vi "test_work(4800).vi"() -> ()   [LabVIEW 2013]
uses:
  IS-95/receiver/4800/Combination device(4800).vi
  IS-95/receiver/common/Path Searcher.vi
  IS-95/transmitter/4800/coding(4800).vi
  IS-95/transmitter/common/interleaver.vi
  IS-95/transmitter/9600/coding(9600).vi
  <vilib>/Analysis/baseanly.llb/A x B.vi
  <vilib>/Analysis/baseanly.llb/Real A x B.vi
  IS-95/receiver/common/Viterbi.vi
  IS-95/receiver/4800/FER(4800).vi
  IS-95/receiver/common/Peak detection.vi
  IS-95/transmitter/4800/syndrom(4800).vi
  IS-95/transmitter/9600/syndrom(9600).vi
  IS-95/receiver/common/metrics.vi
  <vilib>/Analysis/Matrix/Numeric/Conversions/Array To Matrix.vi
  <vilib>/Analysis/Matrix/Numeric/Conversions/Array To Matrix - RA.vi
  <vilib>/ptbypt/Other Functions.llb/Complex Queue PtByPt.vi
  <vilib>/ptbypt/Time Domain.llb/Peak Detector PtByPt.vi
  IS-95/receiver/4800/Gateway(4800).vi
panel:
  in  "Stop Button":bool
  out "ПЕРЕДАЧА":bool[](array[boolean])
  in  "ПЕРЕДАЧА":u16(ring)=2 items=["0", "1", "2", "3", "4", "5", "6", "7", "8", "9", "10", "11", "12", "13", "14", "15", "16", "17", "18", "19", "20", "21", "22", "23", "24", "25", "26", "27", "28", "29", "30", "31", "32", "33", "34", "35", "36", "37", "38", "39", "40", "41", "42", "43", "44", "45", "46", "47", "48", "49", "50", "51", "52", "53", "54", "55", "56", "57", "58", "59", "60", "61", "62", "63"]
  in  "ПРИЕМ":u16(ring)=2 items=["0", "1", "2", "3", "4", "5", "6", "7", "8", "9", "10", "11", "12", "13", "14", "15", "16", "17", "18", "19", "20", "21", "22", "23", "24", "25", "26", "27", "28", "29", "30", "31", "32", "33", "34", "35", "36", "37", "38", "39", "40", "41", "42", "43", "44", "45", "46", "47", "48", "49", "50", "51", "52", "53", "54", "55", "56", "57", "58", "59", "60", "61", "62", "63"]
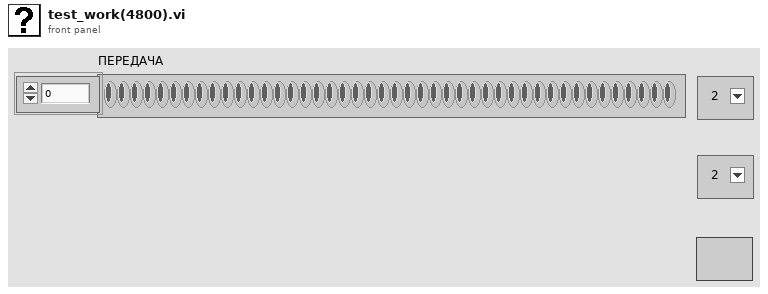
[diagram p1: front panel]
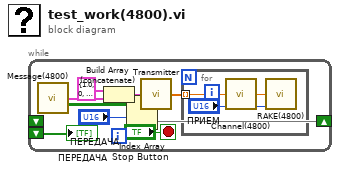
[diagram p0: block diagram]
diagram:
  n1 = while {
    shift-right: [w2] -> _
    shift-left: _ -> [_]
    shift-left: _ -> [w1]
    stop <- "Stop Button" stop-if-true
    n2 = call "Message(4800).vi"() -> ("Channels"=w5:cluster{dbl, i32, bool[], "Type":i32}[], "Message"=w4:bool[][])  [unwired: 14 in]
    n3 = Build Array (concatenate)(cluster{dbl, i32, bool[], "Type":i32} {1.0, 0, [FALSE, FALSE, FALSE, FALSE, FALSE, FALSE, FALSE, FALSE, FALSE, FALSE, FALSE, FALSE, FALSE, FALSE, FALSE, FALSE, FALSE, FALSE, FALSE, FALSE, FALSE, FALSE, FALSE, FALSE, FALSE, FALSE, FALSE, FALSE, FALSE, FALSE, FALSE, FALSE, FALSE, FALSE, FALSE, FALSE, FALSE, FALSE, FALSE, FALSE, FALSE, FALSE, FALSE, FALSE, FALSE, FALSE, FALSE, FALSE, FALSE, FALSE, FALSE, FALSE, FALSE, FALSE, FALSE, FALSE, FALSE, FALSE, FALSE, FALSE, FALSE, FALSE, FALSE, FALSE, FALSE, FALSE, FALSE, FALSE, FALSE, FALSE, FALSE, FALSE, FALSE, FALSE, FALSE, FALSE, FALSE, FALSE, FALSE, FALSE], "Type"=80} ("Frame(PICH) 2"), w5) -> (w8:cluster{dbl, i32, bool[], "Type":i32}[])
    n4 = Index Array(array=w4, index (row)="ПЕРЕДАЧА") -> (element=w2:bool[])  [unwired: 1 in]
    n5 = call "Transmitter.vi"("CHANNELS"=w8) -> ("x + iy"=w7:cdb[])  [unwired: 14 in]
    n6 = for {
      tunnel: w7 -> [w11] mode=indexing
      n7 = call "Channel(4800).vi"("Выборка\nс передатчика"=w11) -> ("Выборка \nс канала"=w10:cdb)  [unwired: 14 in]
      n8 = call "RAKE(4800).vi"("ВЫБОРКА \nОГИБАЮЩЕЙ 2"=w10, "Номер\nканала"="ПРИЕМ") -> ()  [unwired: 14 in]
    }
    "ПЕРЕДАЧА" <- w1
  }
